vi "Project-SmartHome.vi"() -> ()   [LabVIEW 2013] (continued)
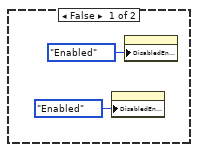
[diagram p2: hidden frame]
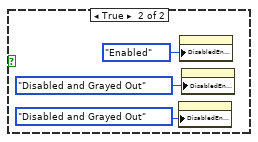
[diagram p3: hidden frame]
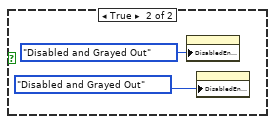
[diagram p4: hidden frame]
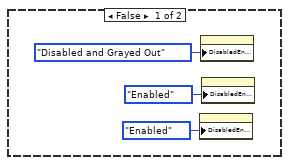
[diagram p5: hidden frame]
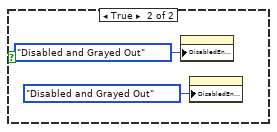
[diagram p6: hidden frame]
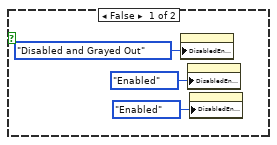
[diagram p7: hidden frame]
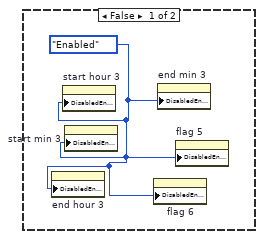
[diagram p8: hidden frame]
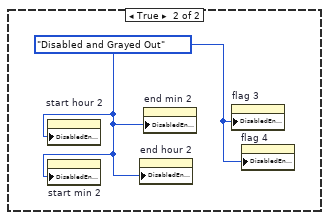
[diagram p9: hidden frame]
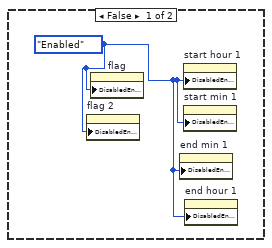
[diagram p10: hidden frame]
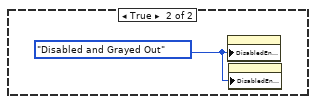
[diagram p11: hidden frame]
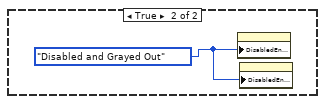
[diagram p12: hidden frame]
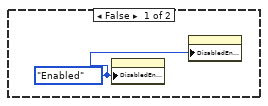
[diagram p13: hidden frame]
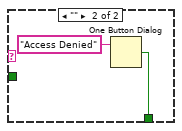
[diagram p15: hidden frame]
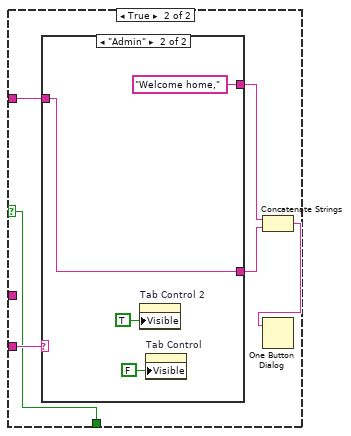
[diagram p16: hidden frame]
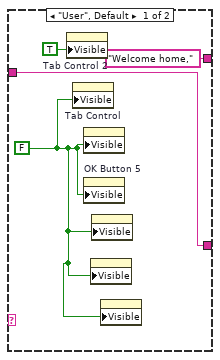
[diagram p17: hidden frame]
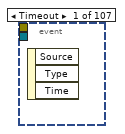
[diagram p18: hidden frame]
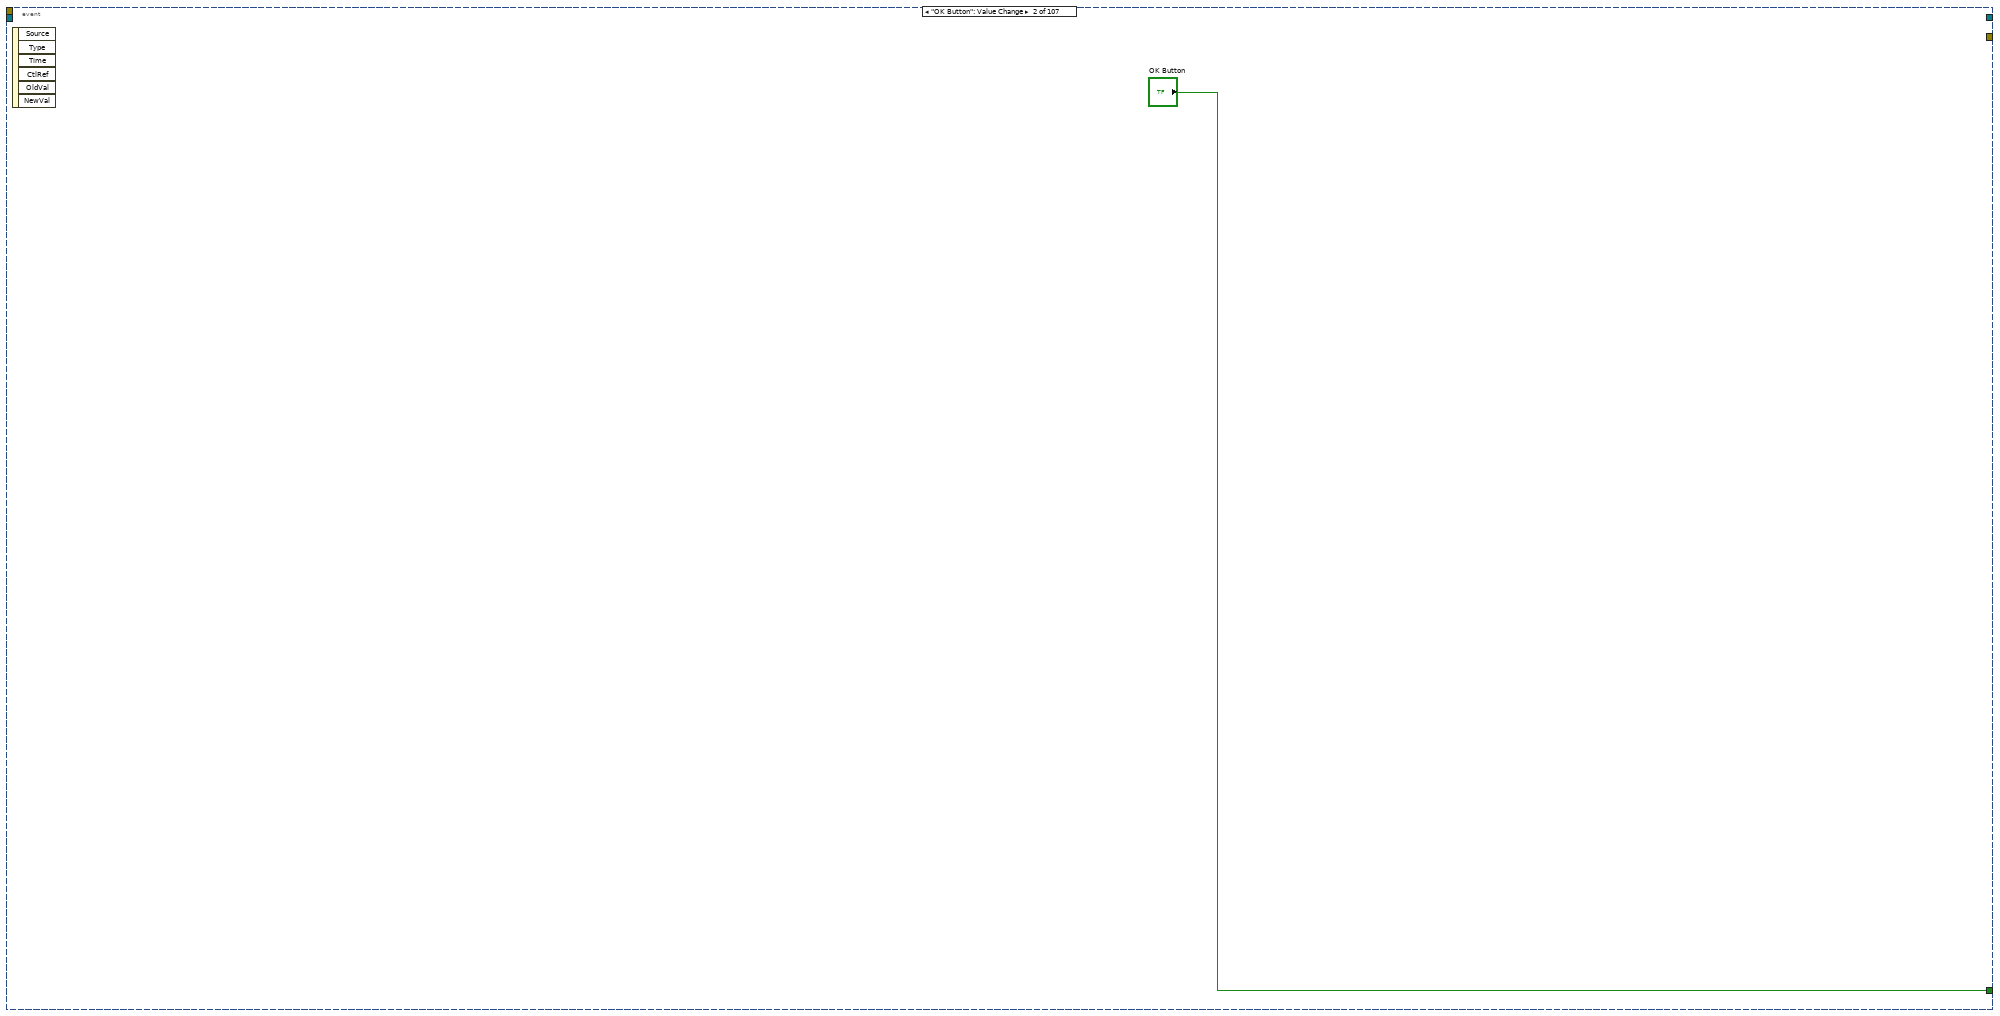
[diagram p19: hidden frame]
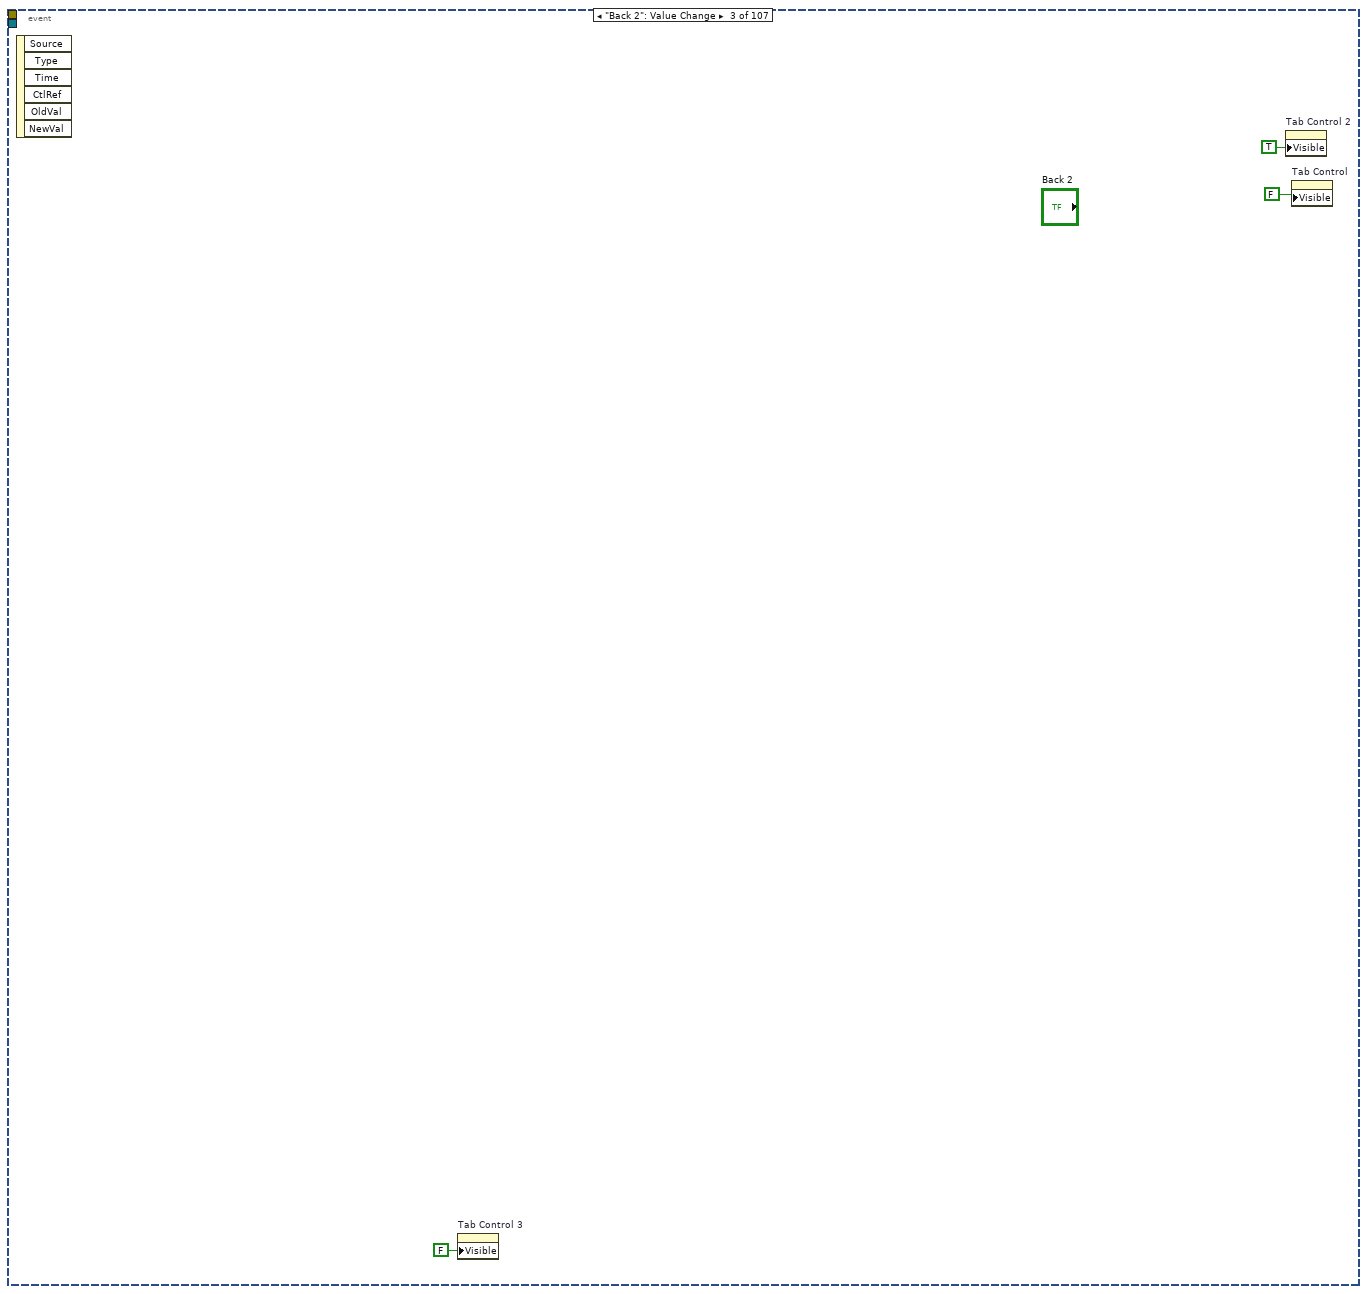
[diagram p20: hidden frame]
        n994 = Bundle("?", 1.0) -> (w2993:cluster{bool, dbl})  [unwired: 1 in]
        n995 = Type Cast(x=w2993) -> (*(type *) &x=w2994:string)  [unwired: 1 in]
        n996 = TCP Write(connection ID=w2987, data in=w2994, error in (no error)=w2988) -> (connection ID out=w2996:refnum<k5>, error out=w2995:errorcluster)  [unwired: 1 in, 1 out]
      }
      event "OK Button 5": Value Change {
        n997 = event-data() -> ()  [unwired: 1 in, 6 out]
        n998 = Type Cast(x=0.0) -> (*(type *) &x=w2997:string)  [unwired: 1 in]
        n999 = TCP Write(connection ID=w3000, data in=w2997, error in (no error)=w3001) -> (connection ID out=w2999:refnum<k5>, error out=w2998:errorcluster)  [unwired: 1 in, 1 out]
        n1000 = Bundle("OK Button 5"="OK Button 5", 2.0) -> (w3007:cluster{"OK Button 5":bool, dbl})  [unwired: 1 in]
        n1001 = Type Cast(x=w3007) -> (*(type *) &x=w3008:string)  [unwired: 1 in]
        n1002 = TCP Write(connection ID=w2999, data in=w3008, error in (no error)=w2998) -> (connection ID out=w3004:refnum<k5>, error out=w3003:errorcluster)  [unwired: 1 in, 1 out]
      }
      event Value Change {
        n1003 = event-data() -> ()  [unwired: 1 in, 6 out]
        n1004 = Add(x=u16 1, y="start hour 1") -> (x+y=w3014:u16)
        n1005 = To Double Precision Float(number=w3014) -> (double precision float=w3026:dbl)
        n1006 = To Double Precision Float(number="start min 1") -> (double precision float=w3025:dbl)
        n1007 = Type Cast(x=3.0) -> (*(type *) &x=w3032:string)  [unwired: 1 in]
        n1008 = TCP Write(connection ID=w3028, data in=w3032, error in (no error)=w3027) -> (connection ID out=w3029:refnum<k5>, error out=w3033:errorcluster)  [unwired: 1 in, 1 out]
        n1009 = Add(x="end hour 1", y=u16 1) -> (x+y=w3012:u16)
        n1010 = To Double Precision Float(number="end min 1") -> (double precision float=w3018:dbl)
        n1011 = To Double Precision Float(number=w3012) -> (double precision float=w3017:dbl)
        n1012 = To Double Precision Float(number="flag") -> (double precision float=w3020:dbl)
        n1013 = To Double Precision Float(number="flag 2") -> (double precision float=w3022:dbl)
        n1014 = Bundle(w3026, w3025, w3017, w3018, w3020, w3022, 1, "?") -> (w3035:cluster{dbl, dbl, dbl, dbl, dbl, dbl, i32, bool})  [unwired: 1 in]
        n1015 = Type Cast(x=w3035) -> (*(type *) &x=w3036:string)  [unwired: 1 in]
        n1016 = TCP Write(connection ID=w3029, data in=w3036, error in (no error)=w3033) -> (connection ID out=w3030:refnum<k5>, error out=w3031:errorcluster)  [unwired: 1 in, 1 out]
      }
      event Value Change {
        n1017 = event-data() -> ()  [unwired: 1 in, 6 out]
        n1018 = Add(x=u16 1, y="start hour 2") -> (x+y=w3048:u16)
        n1019 = To Double Precision Float(number=w3048) -> (double precision float=w3056:dbl)
        n1020 = To Double Precision Float(number="start min 2") -> (double precision float=w3055:dbl)
        n1021 = Add(x="end hour 2", y=u16 1) -> (x+y=w3047:u16)
        n1022 = To Double Precision Float(number="end min 2") -> (double precision float=w3051:dbl)
        n1023 = To Double Precision Float(number=w3047) -> (double precision float=w3050:dbl)
        n1024 = Type Cast(x=3.0) -> (*(type *) &x=w3062:string)  [unwired: 1 in]
        n1025 = TCP Write(connection ID=w3058, data in=w3062, error in (no error)=w3057) -> (connection ID out=w3061:refnum<k5>, error out=w3063:errorcluster)  [unwired: 1 in, 1 out]
        n1026 = To Double Precision Float(number="flag 3") -> (double precision float=w3053:dbl)
        n1027 = To Double Precision Float(number="flag 4") -> (double precision float=w3054:dbl)
        n1028 = Bundle(w3056, w3055, w3050, w3051, w3053, w3054, 2, "?") -> (w3039:cluster{dbl, dbl, dbl, dbl, dbl, dbl, i32, bool})  [unwired: 1 in]
        n1029 = Type Cast(x=w3039) -> (*(type *) &x=w3038:string)  [unwired: 1 in]
        n1030 = TCP Write(connection ID=w3061, data in=w3038, error in (no error)=w3063) -> (connection ID out=w3059:refnum<k5>, error out=w3060:errorcluster)  [unwired: 1 in, 1 out]
      }
      event Value Change {
        n1031 = event-data() -> ()  [unwired: 1 in, 6 out]
        n1032 = Add(x=u16 1, y="start hour 3") -> (x+y=w3078:u16)
        n1033 = To Double Precision Float(number=w3078) -> (double precision float=w3085:dbl)
        n1034 = To Double Precision Float(number="start min 3") -> (double precision float=w3084:dbl)
        n1035 = Add(x="end hour 3", y=u16 1) -> (x+y=w3077:u16)
        n1036 = To Double Precision Float(number="end min 3") -> (double precision float=w3081:dbl)
        n1037 = To Double Precision Float(number=w3077) -> (double precision float=w3080:dbl)
        n1038 = Type Cast(x=3.0) -> (*(type *) &x=w3074:string)  [unwired: 1 in]
        n1039 = TCP Write(connection ID=w3088, data in=w3074, error in (no error)=w3087) -> (connection ID out=w3091:refnum<k5>, error out=w3092:errorcluster)  [unwired: 1 in, 1 out]
        n1040 = To Double Precision Float(number="flag 5") -> (double precision float=w3082:dbl)
        n1041 = To Double Precision Float(number="flag 6") -> (double precision float=w3083:dbl)
        n1042 = Bundle(w3085, w3084, w3080, w3081, w3082, w3083, 3, "?") -> (w3075:cluster{dbl, dbl, dbl, dbl, dbl, dbl, i32, bool})  [unwired: 1 in]
        n1043 = Type Cast(x=w3075) -> (*(type *) &x=w3073:string)  [unwired: 1 in]
        n1044 = TCP Write(connection ID=w3091, data in=w3073, error in (no error)=w3092) -> (connection ID out=w3089:refnum<k5>, error out=w3090:errorcluster)  [unwired: 1 in, 1 out]
      }
      event Value Change {
        # "Air conditional menu"
        n1045 = event-data() -> ()  [unwired: 1 in, 6 out]
        n1046 = property on="Tab Control" class="TabCtl (strict)"("Visible"=FALSE) -> ()  [unwired: 2 in, 2 out]
        n1047 = property on="Tab Control 2" class="TabCtl (strict)"("Visible"=FALSE) -> ()  [unwired: 2 in, 2 out]
        n1048 = property on="Tab Control 3" class="TabCtl (strict)"("Visible"=FALSE) -> ()  [unwired: 2 in, 2 out]
        n1049 = property on="Tab Control 4" class="TabCtl (strict)"("Visible"=FALSE) -> ()  [unwired: 2 in, 2 out]
        n1050 = property on="Tab Control 5" class="TabCtl (strict)"("Visible"=FALSE) -> ()  [unwired: 2 in, 2 out]
        n1051 = property on="Tab Control 13" class="TabCtl (strict)"("Visible"=FALSE) -> ()  [unwired: 2 in, 2 out]
        n1052 = property on="Tab Control 14" class="TabCtl (strict)"("Visible"=FALSE) -> ()  [unwired: 2 in, 2 out]
        n1053 = property on="Tab Control 11" class="TabCtl (strict)"("Visible"=FALSE) -> ()  [unwired: 2 in, 2 out]
        n1054 = property on="Tab Control 6" class="TabCtl (strict)"("Visible"=FALSE) -> ()  [unwired: 2 in, 2 out]
        n1055 = property on="Tab Control 10" class="TabCtl (strict)"("Visible"=FALSE) -> ()  [unwired: 2 in, 2 out]
        n1056 = property on="Tab Control 7" class="TabCtl (strict)"("Visible"=FALSE) -> ()  [unwired: 2 in, 2 out]
        n1057 = property on="Tab Control 12" class="TabCtl (strict)"("Visible"=FALSE) -> ()  [unwired: 2 in, 2 out]
        n1058 = property on="Tab Control 8" class="TabCtl (strict)"("Visible"=FALSE) -> ()  [unwired: 2 in, 2 out]
        n1059 = property on="Tab Control 9" class="TabCtl (strict)"("Visible"=FALSE) -> ()  [unwired: 2 in, 2 out]
        n1060 = property on="Tab Control 15" class="TabCtl (strict)"("Visible"=FALSE) -> ()  [unwired: 2 in, 2 out]
        n1061 = property on="Tab Control 16" class="TabCtl (strict)"("Visible"=FALSE) -> ()  [unwired: 2 in, 2 out]
        n1062 = property on="Tab Control 17" class="TabCtl (strict)"("Visible"=FALSE) -> ()  [unwired: 2 in, 2 out]
        n1063 = property on="Tab Control 21" class="TabCtl (strict)"("Visible"=FALSE) -> ()  [unwired: 2 in, 2 out]
        n1064 = property on="Tab Control 18" class="TabCtl (strict)"("Visible"=FALSE) -> ()  [unwired: 2 in, 2 out]
        n1065 = property on="Tab Control 24" class="TabCtl (strict)"("Visible"=FALSE) -> ()  [unwired: 2 in, 2 out]
        n1066 = property on="Tab Control 19" class="TabCtl (strict)"("Visible"=TRUE) -> ()  [unwired: 2 in, 2 out]
        n1067 = property on="Tab Control 22" class="TabCtl (strict)"("Visible"=FALSE) -> ()  [unwired: 2 in, 2 out]
      }
      event "OK Button 6": Value Change {
        n1068 = event-data() -> ()  [unwired: 1 in, 6 out]
        n1069 = Type Cast(x=0.0) -> (*(type *) &x=w3120:string)  [unwired: 1 in]
        n1070 = TCP Write(connection ID=w3118, data in=w3120, error in (no error)=w3119) -> (connection ID out=w3117:refnum<k5>, error out=w3116:errorcluster)  [unwired: 1 in, 1 out]
        n1071 = Bundle("OK Button 6"="OK Button 6", 5.0) -> (w3125:cluster{"OK Button 6":bool, dbl})  [unwired: 1 in]
        n1072 = Type Cast(x=w3125) -> (*(type *) &x=w3126:string)  [unwired: 1 in]
        n1073 = TCP Write(connection ID=w3117, data in=w3126, error in (no error)=w3116) -> (connection ID out=w3122:refnum<k5>, error out=w3123:errorcluster)  [unwired: 1 in, 1 out]
      }
      event Value Change {
        # "Air conditional - Master room"
        n1074 = event-data() -> ()  [unwired: 1 in, 6 out]
        n1075 = property on="Tab Control 19" class="TabCtl (strict)"("Visible"=FALSE) -> ()  [unwired: 2 in, 2 out]
        n1076 = property on="Tab Control" class="TabCtl (strict)"("Visible"=FALSE) -> ()  [unwired: 2 in, 2 out]
        n1077 = property on="Tab Control 2" class="TabCtl (strict)"("Visible"=FALSE) -> ()  [unwired: 2 in, 2 out]
        n1078 = property on="Tab Control 3" class="TabCtl (strict)"("Visible"=FALSE) -> ()  [unwired: 2 in, 2 out]
        n1079 = property on="Tab Control 4" class="TabCtl (strict)"("Visible"=FALSE) -> ()  [unwired: 2 in, 2 out]
        n1080 = property on="Tab Control 5" class="TabCtl (strict)"("Visible"=FALSE) -> ()  [unwired: 2 in, 2 out]
        n1081 = property on="Tab Control 13" class="TabCtl (strict)"("Visible"=FALSE) -> ()  [unwired: 2 in, 2 out]
        n1082 = property on="Tab Control 14" class="TabCtl (strict)"("Visible"=FALSE) -> ()  [unwired: 2 in, 2 out]
        n1083 = property on="Tab Control 11" class="TabCtl (strict)"("Visible"=FALSE) -> ()  [unwired: 2 in, 2 out]
        n1084 = property on="Tab Control 6" class="TabCtl (strict)"("Visible"=FALSE) -> ()  [unwired: 2 in, 2 out]
        n1085 = property on="Tab Control 10" class="TabCtl (strict)"("Visible"=FALSE) -> ()  [unwired: 2 in, 2 out]
        n1086 = property on="Tab Control 7" class="TabCtl (strict)"("Visible"=FALSE) -> ()  [unwired: 2 in, 2 out]
        n1087 = property on="Tab Control 12" class="TabCtl (strict)"("Visible"=FALSE) -> ()  [unwired: 2 in, 2 out]
        n1088 = property on="Tab Control 8" class="TabCtl (strict)"("Visible"=FALSE) -> ()  [unwired: 2 in, 2 out]
        n1089 = property on="Tab Control 9" class="TabCtl (strict)"("Visible"=FALSE) -> ()  [unwired: 2 in, 2 out]
        n1090 = property on="Tab Control 15" class="TabCtl (strict)"("Visible"=FALSE) -> ()  [unwired: 2 in, 2 out]
        n1091 = property on="Tab Control 16" class="TabCtl (strict)"("Visible"=FALSE) -> ()  [unwired: 2 in, 2 out]
        n1092 = property on="Tab Control 17" class="TabCtl (strict)"("Visible"=FALSE) -> ()  [unwired: 2 in, 2 out]
        n1093 = property on="Tab Control 24" class="TabCtl (strict)"("Visible"=FALSE) -> ()  [unwired: 2 in, 2 out]
        n1094 = property on="Tab Control 18" class="TabCtl (strict)"("Visible"=FALSE) -> ()  [unwired: 2 in, 2 out]
        n1095 = property on="Tab Control 21" class="TabCtl (strict)"("Visible"=FALSE) -> ()  [unwired: 2 in, 2 out]
        n1096 = property on="Tab Control 19" class="TabCtl (strict)"("Visible"=FALSE) -> ()  [unwired: 2 in, 2 out]
        n1097 = property on="Tab Control 22" class="TabCtl (strict)"("Visible"=TRUE) -> ()  [unwired: 2 in, 2 out]
      }
      event Value Change {
        # "Air conditional - Bedroom 1"
        n1098 = event-data() -> ()  [unwired: 1 in, 6 out]
        n1099 = property on="Tab Control" class="TabCtl (strict)"("Visible"=FALSE) -> ()  [unwired: 2 in, 2 out]
        n1100 = property on="Tab Control 2" class="TabCtl (strict)"("Visible"=FALSE) -> ()  [unwired: 2 in, 2 out]
        n1101 = property on="Tab Control 3" class="TabCtl (strict)"("Visible"=FALSE) -> ()  [unwired: 2 in, 2 out]
        n1102 = property on="Tab Control 4" class="TabCtl (strict)"("Visible"=FALSE) -> ()  [unwired: 2 in, 2 out]
        n1103 = property on="Tab Control 5" class="TabCtl (strict)"("Visible"=FALSE) -> ()  [unwired: 2 in, 2 out]
        n1104 = property on="Tab Control 11" class="TabCtl (strict)"("Visible"=FALSE) -> ()  [unwired: 2 in, 2 out]
        n1105 = property on="Tab Control 6" class="TabCtl (strict)"("Visible"=FALSE) -> ()  [unwired: 2 in, 2 out]
        n1106 = property on="Tab Control 10" class="TabCtl (strict)"("Visible"=FALSE) -> ()  [unwired: 2 in, 2 out]
        n1107 = property on="Tab Control 13" class="TabCtl (strict)"("Visible"=FALSE) -> ()  [unwired: 2 in, 2 out]
        n1108 = property on="Tab Control 7" class="TabCtl (strict)"("Visible"=FALSE) -> ()  [unwired: 2 in, 2 out]
        n1109 = property on="Tab Control 12" class="TabCtl (strict)"("Visible"=FALSE) -> ()  [unwired: 2 in, 2 out]
        n1110 = property on="Tab Control 8" class="TabCtl (strict)"("Visible"=FALSE) -> ()  [unwired: 2 in, 2 out]
        n1111 = property on="Tab Control 9" class="TabCtl (strict)"("Visible"=FALSE) -> ()  [unwired: 2 in, 2 out]
        n1112 = property on="Tab Control 21" class="TabCtl (strict)"("Visible"=FALSE) -> ()  [unwired: 2 in, 2 out]
        n1113 = property on="Tab Control 22" class="TabCtl (strict)"("Visible"=FALSE) -> ()  [unwired: 2 in, 2 out]
        n1114 = property on="Tab Control 23" class="TabCtl (strict)"("Visible"=TRUE) -> ()  [unwired: 2 in, 2 out]
        n1115 = property on="Tab Control 24" class="TabCtl (strict)"("Visible"=FALSE) -> ()  [unwired: 2 in, 2 out]
        n1116 = property on="Tab Control 14" class="TabCtl (strict)"("Visible"=FALSE) -> ()  [unwired: 2 in, 2 out]
        n1117 = property on="Tab Control 15" class="TabCtl (strict)"("Visible"=FALSE) -> ()  [unwired: 2 in, 2 out]
        n1118 = property on="Tab Control 20" class="TabCtl (strict)"("Visible"=FALSE) -> ()  [unwired: 2 in, 2 out]
        n1119 = property on="Tab Control 16" class="TabCtl (strict)"("Visible"=FALSE) -> ()  [unwired: 2 in, 2 out]
        n1120 = property on="Tab Control 17" class="TabCtl (strict)"("Visible"=FALSE) -> ()  [unwired: 2 in, 2 out]
        n1121 = property on="Tab Control 18" class="TabCtl (strict)"("Visible"=FALSE) -> ()  [unwired: 2 in, 2 out]
        n1122 = property on="Tab Control 19" class="TabCtl (strict)"("Visible"=FALSE) -> ()  [unwired: 2 in, 2 out]
      }
      event "OK Button 7": Value Change {
        n1123 = event-data() -> ()  [unwired: 1 in, 6 out]
        n1124 = Type Cast(x=0.0) -> (*(type *) &x=w3179:string)  [unwired: 1 in]
        n1125 = TCP Write(connection ID=w3177, data in=w3179, error in (no error)=w3174) -> (connection ID out=w3176:refnum<k5>, error out=w3175:errorcluster)  [unwired: 1 in, 1 out]
        n1126 = Bundle("OK Button 7"="OK Button 7", 6.0) -> (w3184:cluster{"OK Button 7":bool, dbl})  [unwired: 1 in]
        n1127 = Type Cast(x=w3184) -> (*(type *) &x=w3185:string)  [unwired: 1 in]
        n1128 = TCP Write(connection ID=w3176, data in=w3185, error in (no error)=w3175) -> (connection ID out=w3181:refnum<k5>, error out=w3182:errorcluster)  [unwired: 1 in, 1 out]
      }
      event "OK Button 8": Value Change {
        n1129 = event-data() -> ()  [unwired: 1 in, 6 out]
        n1130 = Type Cast(x=0.0) -> (*(type *) &x=w3191:string)  [unwired: 1 in]
        n1131 = TCP Write(connection ID=w3187, data in=w3191, error in (no error)=w3186) -> (connection ID out=w3188:refnum<k5>, error out=w3189:errorcluster)  [unwired: 1 in, 1 out]
        n1132 = Bundle("OK Button 8"="OK Button 8", 7.0) -> (w3196:cluster{"OK Button 8":bool, dbl})  [unwired: 1 in]
        n1133 = Type Cast(x=w3196) -> (*(type *) &x=w3197:string)  [unwired: 1 in]
        n1134 = TCP Write(connection ID=w3188, data in=w3197, error in (no error)=w3189) -> (connection ID out=w3193:refnum<k5>, error out=w3194:errorcluster)  [unwired: 1 in, 1 out]
      }
      event "OK Button 9": Value Change {
        n1135 = event-data() -> ()  [unwired: 1 in, 6 out]
        n1136 = Type Cast(x=0.0) -> (*(type *) &x=w3198:string)  [unwired: 1 in]
        n1137 = TCP Write(connection ID=w3200, data in=w3198, error in (no error)=w3199) -> (connection ID out=w3201:refnum<k5>, error out=w3202:errorcluster)  [unwired: 1 in, 1 out]
        n1138 = Bundle("OK Button 9"="OK Button 9", 10.0) -> (w3208:cluster{"OK Button 9":bool, dbl})  [unwired: 1 in]
        n1139 = Type Cast(x=w3208) -> (*(type *) &x=w3209:string)  [unwired: 1 in]
        n1140 = TCP Write(connection ID=w3201, data in=w3209, error in (no error)=w3202) -> (connection ID out=w3205:refnum<k5>, error out=w3206:errorcluster)  [unwired: 1 in, 1 out]
      }
      event "OK Button 10": Value Change {
        n1141 = event-data() -> ()  [unwired: 1 in, 6 out]
        n1142 = Type Cast(x=0.0) -> (*(type *) &x=w3210:string)  [unwired: 1 in]
        n1143 = TCP Write(connection ID=w3214, data in=w3210, error in (no error)=w3213) -> (connection ID out=w3212:refnum<k5>, error out=w3211:errorcluster)  [unwired: 1 in, 1 out]
        n1144 = Bundle("OK Button 10"="OK Button 10", 11.0) -> (w3220:cluster{"OK Button 10":bool, dbl})  [unwired: 1 in]
        n1145 = Type Cast(x=w3220) -> (*(type *) &x=w3221:string)  [unwired: 1 in]
        n1146 = TCP Write(connection ID=w3212, data in=w3221, error in (no error)=w3211) -> (connection ID out=w3217:refnum<k5>, error out=w3218:errorcluster)  [unwired: 1 in, 1 out]
      }
    }
    n1147 = case shown="True" w28 {
      frame False {
        w75 = T1."Enabled" ("Disabled")
        n1148 = property class="Slide (strict)"("DisabledEnum"=w75) -> ()  [unwired: 2 in, 2 out]
        n1149 = property class="Str"("DisabledEnum"=w75) -> ()  [unwired: 2 in, 2 out]
      }
      frame True {
        w76 = T1."Disabled and Grayed Out" ("Disabled")
        n1150 = property class="Slide (strict)"("DisabledEnum"=w76) -> ()  [unwired: 2 in, 2 out]
        n1151 = property class="Str"("DisabledEnum"=w76) -> ()  [unwired: 2 in, 2 out]
      }
    }
    n1152 = case shown="False" w27 {
      frame False {
        w73 = T1."Enabled" ("Disabled")
        n1153 = property class="Slide (strict)"("DisabledEnum"=w73) -> ()  [unwired: 2 in, 2 out]
        n1154 = property class="Str"("DisabledEnum"=w73) -> ()  [unwired: 2 in, 2 out]
      }
      frame True {
        w74 = T1."Disabled and Grayed Out" ("Disabled")
        n1155 = property class="Slide (strict)"("DisabledEnum"=w74) -> ()  [unwired: 2 in, 2 out]
        n1156 = property class="Str"("DisabledEnum"=w74) -> ()  [unwired: 2 in, 2 out]
      }
    }
    n1157 = case shown="True" w25 {
      frame False {
        w69 = T1."Enabled" ("Disabled")
        n1158 = property on="flag 2" class="Ring (strict)"("DisabledEnum"=w69) -> ()  [unwired: 2 in, 2 out]
        n1159 = property on="flag" class="Ring (strict)"("DisabledEnum"=w69) -> ()  [unwired: 2 in, 2 out]
        n1160 = property on="end min 1" class="Ring (strict)"("DisabledEnum"=w69) -> ()  [unwired: 2 in, 2 out]
        n1161 = property on="start hour 1" class="Ring (strict)"("DisabledEnum"=w69) -> ()  [unwired: 2 in, 2 out]
        n1162 = property on="start min 1" class="Ring (strict)"("DisabledEnum"=w69) -> ()  [unwired: 2 in, 2 out]
        n1163 = property on="end hour 1" class="Ring (strict)"("DisabledEnum"=w69) -> ()  [unwired: 2 in, 2 out]
      }
      frame True {
        w70 = T1."Disabled and Grayed Out" ("Disabled")
        n1164 = property on="flag 2" class="Ring (strict)"("DisabledEnum"=w70) -> ()  [unwired: 2 in, 2 out]
        n1165 = property on="flag" class="Ring (strict)"("DisabledEnum"=w70) -> ()  [unwired: 2 in, 2 out]
        n1166 = property on="end min 1" class="Ring (strict)"("DisabledEnum"=w70) -> ()  [unwired: 2 in, 2 out]
        n1167 = property on="start hour 1" class="Ring (strict)"("DisabledEnum"=w70) -> ()  [unwired: 2 in, 2 out]
        n1168 = property on="start min 1" class="Ring (strict)"("DisabledEnum"=w70) -> ()  [unwired: 2 in, 2 out]
        n1169 = property on="end hour 1" class="Ring (strict)"("DisabledEnum"=w70) -> ()  [unwired: 2 in, 2 out]
      }
    }
    n1170 = case shown="False" w26 {
      frame False {
        w71 = T1."Enabled" ("Disabled")
        n1171 = property class="Slide (strict)"("DisabledEnum"=w71) -> ()  [unwired: 2 in, 2 out]
        n1172 = property class="Str"("DisabledEnum"=w71) -> ()  [unwired: 2 in, 2 out]
      }
      frame True {
        w72 = T1."Disabled and Grayed Out" ("Disabled")
        n1173 = property class="Slide (strict)"("DisabledEnum"=w72) -> ()  [unwired: 2 in, 2 out]
        n1174 = property class="Str"("DisabledEnum"=w72) -> ()  [unwired: 2 in, 2 out]
      }
    }
    n1175 = case shown="False" w24 {
      frame False {
        w67 = T1."Enabled" ("Disabled")
        n1176 = property on="start hour 2" class="Ring (strict)"("DisabledEnum"=w67) -> ()  [unwired: 2 in, 2 out]
        n1177 = property on="start min 2" class="Ring (strict)"("DisabledEnum"=w67) -> ()  [unwired: 2 in, 2 out]
        n1178 = property on="end hour 2" class="Ring (strict)"("DisabledEnum"=w67) -> ()  [unwired: 2 in, 2 out]
        n1179 = property on="end min 2" class="Ring (strict)"("DisabledEnum"=w67) -> ()  [unwired: 2 in, 2 out]
        n1180 = property on="flag 3" class="Ring (strict)"("DisabledEnum"=w67) -> ()  [unwired: 2 in, 2 out]
        n1181 = property on="flag 4" class="Ring (strict)"("DisabledEnum"=w67) -> ()  [unwired: 2 in, 2 out]
      }
      frame True {
        w68 = T1."Disabled and Grayed Out" ("Disabled")
        n1182 = property on="start hour 2" class="Ring (strict)"("DisabledEnum"=w68) -> ()  [unwired: 2 in, 2 out]
        n1183 = property on="start min 2" class="Ring (strict)"("DisabledEnum"=w68) -> ()  [unwired: 2 in, 2 out]
        n1184 = property on="end hour 2" class="Ring (strict)"("DisabledEnum"=w68) -> ()  [unwired: 2 in, 2 out]
        n1185 = property on="end min 2" class="Ring (strict)"("DisabledEnum"=w68) -> ()  [unwired: 2 in, 2 out]
        n1186 = property on="flag 3" class="Ring (strict)"("DisabledEnum"=w68) -> ()  [unwired: 2 in, 2 out]
        n1187 = property on="flag 4" class="Ring (strict)"("DisabledEnum"=w68) -> ()  [unwired: 2 in, 2 out]
      }
    }
    n1188 = case shown="True" w23 {
      frame False {
        w65 = T1."Enabled" ("Disabled")
        n1189 = property on="end hour 3" class="Ring (strict)"("DisabledEnum"=w65) -> ()  [unwired: 2 in, 2 out]
        n1190 = property on="start hour 3" class="Ring (strict)"("DisabledEnum"=w65) -> ()  [unwired: 2 in, 2 out]
        n1191 = property on="start min 3" class="Ring (strict)"("DisabledEnum"=w65) -> ()  [unwired: 2 in, 2 out]
        n1192 = property on="flag 6" class="Ring (strict)"("DisabledEnum"=w65) -> ()  [unwired: 2 in, 2 out]
        n1193 = property on="end min 3" class="Ring (strict)"("DisabledEnum"=w65) -> ()  [unwired: 2 in, 2 out]
        n1194 = property on="flag 5" class="Ring (strict)"("DisabledEnum"=w65) -> ()  [unwired: 2 in, 2 out]
      }
      frame True {
        w66 = T1."Disabled and Grayed Out" ("Disabled")
        n1195 = property on="end hour 3" class="Ring (strict)"("DisabledEnum"=w66) -> ()  [unwired: 2 in, 2 out]
        n1196 = property on="start hour 3" class="Ring (strict)"("DisabledEnum"=w66) -> ()  [unwired: 2 in, 2 out]
        n1197 = property on="start min 3" class="Ring (strict)"("DisabledEnum"=w66) -> ()  [unwired: 2 in, 2 out]
        n1198 = property on="flag 6" class="Ring (strict)"("DisabledEnum"=w66) -> ()  [unwired: 2 in, 2 out]
        n1199 = property on="end min 3" class="Ring (strict)"("DisabledEnum"=w66) -> ()  [unwired: 2 in, 2 out]
        n1200 = property on="flag 5" class="Ring (strict)"("DisabledEnum"=w66) -> ()  [unwired: 2 in, 2 out]
      }
    }
    n1201 = case shown="True" w34 {
      frame False {
      }
      frame True {
        n1202 = Read from Text File(file (use dialog)=path "C:/Users/kiat/Desktop/password.txt") -> (text=w77:string)  [unwired: 3 in, 3 out]
        n1203 = while {
          border: w77 -> [_]
          stop <- w81 stop-if-true
          n1204 = feedback #7() -> (w88:string)
          n1205 = xnode "Match Regular Expression"("input string"=w88, "regular expression"="\n") -> ("before match"=w87:string, "after match"=w79:string)  [unwired: 4 in, 3 out]
          n1206 = feedback-in #7(w79) -> ()
          n1207 = xnode "Match Regular Expression"("input string"=w87, "regular expression"="-") -> ("before match"=w93:string, "after match"=w86:string)  [unwired: 4 in, 3 out]
          n1208 = xnode "Match Regular Expression"("input string"=w86, "regular expression"=":") -> ("before match"=w84:string, "after match"=w82:string)  [unwired: 4 in, 3 out]
          n1209 = Equal?(x="String", y=w93) -> (x = y?=w90:bool)
          n1210 = Equal?(x=w84, y="String 2") -> (x = y?=w91:bool)
          n1211 = And(x=w90, y=w91) -> (x .and. y?=w83:bool)
          n1212 = case shown="False" w83 {
            selector: w83 -> [w95 w105]
            tunnel: w82 -> [_ w106]
            tunnel: [w97 w105] -> w81
            tunnel: "String" -> [_ w104]
            tunnel: w79 -> [w96 _]
            frame False {
              n1213 = case shown="\"False\", Default" w96 {
                tunnel: [w98 w99] -> w97
                tunnel: w95 -> [w98 _]
                frame "False", Default {
                }
                frame "" {
                  n1214 = One Button Dialog(message="Access Denied") -> (true=w99:bool)  [unwired: 1 in]
                }
              }
            }
            frame True {
              n1215 = case shown="\"Admin\"" w106 {
                tunnel: w104 -> [w108 w112]
                tunnel: [w108 w112] -> w103
                tunnel: ["Welcome home," ("string") "Welcome home," ("string")] -> w102
                frame "User", Default {
                  w110 = FALSE ("Visible")
                  n1216 = property on="Tab Control 2" class="TabCtl (strict)"("Visible"=TRUE) -> ()  [unwired: 2 in, 2 out]
                  n1217 = property on="Tab Control" class="TabCtl (strict)"("Visible"=w110) -> ()  [unwired: 2 in, 2 out]
                  n1218 = property class="Bool"("Visible"=w110) -> ()  [unwired: 2 in, 2 out]
                  n1219 = property on="OK Button 5" class="Bool (strict)"("Visible"=w110) -> ()  [unwired: 2 in, 2 out]
                  n1220 = property class="Bool (strict)"("Visible"=w110) -> ()  [unwired: 2 in, 2 out]
                  n1221 = property class="Bool"("Visible"=w110) -> ()  [unwired: 2 in, 2 out]
                  n1222 = property class="Bool"("Visible"=w110) -> ()  [unwired: 2 in, 2 out]
                }
                frame "Admin" {
                  n1223 = property on="Tab Control 2" class="TabCtl (strict)"("Visible"=TRUE) -> ()  [unwired: 2 in, 2 out]
                  n1224 = property on="Tab Control" class="TabCtl (strict)"("Visible"=FALSE) -> ()  [unwired: 2 in, 2 out]
                }
              }
              n1225 = Concatenate Strings(w102, w103) -> (w101:string)
              n1226 = One Button Dialog(message=w101) -> ()  [unwired: 1 in, 1 out]
            }
          }
        }
      }
    }
    n1227 = local read item#11() -> (w21:bool)
    n1228 = local read item#9() -> (w22:bool)
    n1229 = local read item#5() -> (w20:bool)
    n1230 = case shown="False" w21 {
      frame False {
        n1231 = property class="Bool (strict)"("DisabledEnum"=T1."Enabled" ("Disabled")) -> ()  [unwired: 2 in, 2 out]
        n1232 = property class="Slide (strict)"("DisabledEnum"=T1."Enabled" ("Disabled")) -> ()  [unwired: 2 in, 2 out]
      }
      frame True {
        n1233 = property class="Bool (strict)"("DisabledEnum"=T1."Disabled and Grayed Out" ("Disabled")) -> ()  [unwired: 2 in, 2 out]
        n1234 = property class="Slide (strict)"("DisabledEnum"=T1."Disabled and Grayed Out" ("Disabled")) -> ()  [unwired: 2 in, 2 out]
      }
    }
    n1235 = case shown="True" w22 {
      frame False {
        n1236 = property class="Slide (strict)"("DisabledEnum"=T1."Disabled and Grayed Out" ("Disabled")) -> ()  [unwired: 2 in, 2 out]
        n1237 = property class="Bool (strict)"("DisabledEnum"=T1."Enabled" ("Disabled")) -> ()  [unwired: 2 in, 2 out]
        n1238 = property class="Str"("DisabledEnum"=T1."Enabled" ("Disabled")) -> ()  [unwired: 2 in, 2 out]
      }
      frame True {
        n1239 = property class="Slide (strict)"("DisabledEnum"=T1."Enabled" ("Disabled")) -> ()  [unwired: 2 in, 2 out]
        n1240 = property class="Bool (strict)"("DisabledEnum"=T1."Disabled and Grayed Out" ("Disabled")) -> ()  [unwired: 2 in, 2 out]
        n1241 = property class="Str"("DisabledEnum"=T1."Disabled and Grayed Out" ("Disabled")) -> ()  [unwired: 2 in, 2 out]
      }
    }
    n1242 = case shown="True" w20 {
      frame False {
        n1243 = property class="Str"("DisabledEnum"=T1."Enabled" ("Disabled")) -> ()  [unwired: 2 in, 2 out]
        n1244 = property class="Slide (strict)"("DisabledEnum"=T1."Disabled and Grayed Out" ("Disabled")) -> ()  [unwired: 2 in, 2 out]
        n1245 = property class="Bool (strict)"("DisabledEnum"=T1."Enabled" ("Disabled")) -> ()  [unwired: 2 in, 2 out]
      }
      frame True {
        n1246 = property class="Str"("DisabledEnum"=T1."Disabled and Grayed Out" ("Disabled")) -> ()  [unwired: 2 in, 2 out]
        n1247 = property class="Slide (strict)"("DisabledEnum"=T1."Enabled" ("Disabled")) -> ()  [unwired: 2 in, 2 out]
        n1248 = property class="Bool (strict)"("DisabledEnum"=T1."Disabled and Grayed Out" ("Disabled")) -> ()  [unwired: 2 in, 2 out]
      }
    }
    n1249 = local read item#7() -> (w19:bool)
    n1250 = case shown="False" w19 {
      frame False {
        n1251 = property class="Slide (strict)"("DisabledEnum"=T1."Enabled" ("Disabled")) -> ()  [unwired: 2 in, 2 out]
        n1252 = property class="Bool (strict)"("DisabledEnum"=T1."Enabled" ("Disabled")) -> ()  [unwired: 2 in, 2 out]
      }
      frame True {
        n1253 = property class="Slide (strict)"("DisabledEnum"=T1."Disabled and Grayed Out" ("Disabled")) -> ()  [unwired: 2 in, 2 out]
        n1254 = property class="Bool (strict)"("DisabledEnum"=T1."Disabled and Grayed Out" ("Disabled")) -> ()  [unwired: 2 in, 2 out]
      }
    }
    n1255 = local read item#1() -> (w18:bool)
    n1256 = local read item#3() -> (w17:bool)
    n1257 = case shown="False" w18 {
      frame False {
        n1258 = property class="Bool (strict)"("DisabledEnum"=T1."Enabled" ("Disabled")) -> ()  [unwired: 2 in, 2 out]
        n1259 = property class="Str"("DisabledEnum"=T1."Enabled" ("Disabled")) -> ()  [unwired: 2 in, 2 out]
        n1260 = property class="Slide (strict)"("DisabledEnum"=T1."Disabled and Grayed Out" ("Disabled")) -> ()  [unwired: 2 in, 2 out]
      }
      frame True {
        n1261 = property class="Str"("DisabledEnum"=T1."Disabled and Grayed Out" ("Disabled")) -> ()  [unwired: 2 in, 2 out]
        n1262 = property class="Slide (strict)"("DisabledEnum"=T1."Enabled" ("Disabled")) -> ()  [unwired: 2 in, 2 out]
        n1263 = property class="Bool (strict)"("DisabledEnum"=T1."Disabled and Grayed Out" ("Disabled")) -> ()  [unwired: 2 in, 2 out]
      }
    }
    n1264 = case shown="True" w17 {
      frame False {
        n1265 = property class="Bool (strict)"("DisabledEnum"=T1."Enabled" ("Disabled")) -> ()  [unwired: 2 in, 2 out]
        n1266 = property class="Slide (strict)"("DisabledEnum"=T1."Enabled" ("Disabled")) -> ()  [unwired: 2 in, 2 out]
      }
      frame True {
        n1267 = property class="Bool (strict)"("DisabledEnum"=T1."Disabled and Grayed Out" ("Disabled")) -> ()  [unwired: 2 in, 2 out]
        n1268 = property class="Slide (strict)"("DisabledEnum"=T1."Disabled and Grayed Out" ("Disabled")) -> ()  [unwired: 2 in, 2 out]
      }
    }
  }
  n1269 = Read from Text File(file (use dialog)=path "C:/Users/kiat/Desktop/password.txt") -> (text=w1:string)  [unwired: 3 in, 3 out]
  n1270 = while {
    border: w1 -> [_]
    stop <- w3230 stop-if-true
    n1271 = feedback #8() -> (w3234:string)
    n1272 = xnode "Match Regular Expression"("input string"=w3234, "regular expression"="\n") -> ("before match"=w3233:string, "after match"=w3232:string)  [unwired: 4 in, 3 out]
    n1273 = feedback-in #8(w3232) -> ()
    n1274 = xnode "Match Regular Expression"("input string"=w3233, "regular expression"="-") -> ("before match"=w3229:string, "after match"=w3228:string)  [unwired: 4 in, 3 out]
    n1275 = Equal?(x=w3232, y="") -> (x = y?=w3230:bool)
    n1276 = xnode "Match Regular Expression"("input string"=w3228, "regular expression"=":") -> ("before match"=w3225:string, "after match"=w3226:string)  [unwired: 4 in, 3 out]
    n1277 = local read "Table Control"() -> (w3222:string[][])
    n1278 = Build Array(w3229, w3225, w3226) -> (w3224:string[])
    n1279 = Insert Into Array(array=w3222, new element=w3224) -> (w3223:string[][])  [unwired: 2 in]
    n1280 = local write "Table Control"(w3223) -> ()
  }
  n1281 = TCP Close Connection(connection ID=w10, error in (no error)=w7) -> (error out=w11:errorcluster)  [unwired: 1 in, 1 out]
  n1282 = call <vilib>:"Clear Errors.vi"("error in (no error)"=w11) -> ()  [unwired: 6 in, 1 out]
  "Table Control" <- string[][] [] ("Table Control")
  "Numeric" <- 1.0
